vi "Alyssa_GlueLines.vi"() -> ()   [LabVIEW 2016]
uses:
  C:/Users/Aerotech/Documents/BNLStaveAssembly-blueprint/Bin/Aerotech.A3200.dll
  BNLStaveAssembly-blueprint/Bin/Aerotech.A3200.dll
  <vilib>/vision/Image Controls.llb/IMAQ Image.ctl
  <vilib>/LabVIEW Interface for Arduino/Type Defs/Arduino Resource.ctl
  <vilib>/LabVIEW Interface for Arduino/Type Defs/Board Type.ctl
  <vilib>/LabVIEW Interface for Arduino/Type Defs/Pin Mode.ctl
  <vilib>/LabVIEW Interface for Arduino/LabVIEW Interface for Arduino.lvlib
panel:
  out "Module Start":T1
  in  "How many SHORT lines? (actual # will be x2)":i32
  out "XYZ .NET Refnum out 2":refnum<k24>
  in  "y dist (mm)":dbl
  in  "How many lines? (actual # will be x2)":i32
  out "XYZ .NET Refnum out":refnum<k24>
  in  "?":T2(tab)
  in  "Module corner coordinates":T3={"X [mm]"=-325.4922095457569, "Y [mm]"=111.42987050829626, "Z [mm] "=34.99996599632762}
  in  "Axis speeds (mm/s)":T4={"vX [mm]"=49.0, "vY [mm]"=49.0, "vZ [mm] "=49.0}
  in  "Home?":bool
  in  "Lowest Z Position":dbl=38.0
  out "Arduino Resource":T5={"VISA resource"="GlueCTRL", "Board Type"=enum."Uno", "Connection Type"=enum."USB / Serial", "Bytes Per Packet (15)"=15}
  in  "Digital I/O Pin":u8=7
  in  "XYZ Stage Control":refnum<k24>
  in  "Testing?":bool
  out "Difference camera/syringe in X":dbl=-133.03368290747076
  out "Difference camera/syringe in y":dbl=-2.170984960815403
  in  "um/pix resolution":dbl=1.58
  in  "Image Feed":T7=refnum
  in  "Path to save collected images":path=path "C:/Users/Aerotech/cernbox/BNL/Stave Assembly Records/2017-06-12/3"
  in  "Estimate distance y":dbl
  in  "Estimate distance x":dbl=130.0
  in  "Lowest Z position Calibration":dbl=17.0
  out "Final Position":T1={"Final X"=-325.49379764644783, "Final Y"=23.533617154160947, "Final Z"=34.99956596392527}
  out "error out":errorcluster={"status"=FALSE, "code"=1073676418, "source"="VISA Close in GlueSingleModule(SubVI).vi->2_VisualizeModulePositioning2.vi->VMP_TestStand.vi"}
  in  "error in":errorcluster
  # "Timers (ms)"
  # "Overview: This takes a pattern of zeroes/ones (.csv file) as well as the start coordinates of the top left corner of a module and places dots of glue  \nRequirements: NI Arduino dependencies\nInstructions: Select a .csv file (ones indicate regions for glue) as well as a starting coordinate (this is default to the top left corner of the module spacer). You \ncan also input axis speeds (default to maximum) and module lengths and widths (default to 90 mm) which are the widths of the module to which you want to \nplace glue. Lastly, one can choose to Home the stage here and can select the lowest position in Z. The default is that the stage moves down 2-3 mm in Z \nwhile dispensing.  The Arduino inputs are default and simply allow the LabView program to drigger the Arduino (which sends a signal to the dispenser). The \nprogram signals to dispense air- all other parameters such as length of dispensing (default: 350 millisec), pressure (default: 48 psi), and vacuum pressure \n(default: 7.8 psi) are set on the dispenser itself. The defaults are highly recommended here."
  # "Positioning Inputs"
  # "Arduino Inputs"
types:
  T1 = cluster{"Final X":dbl, "Final Y":dbl, "Final Z":dbl}
  T2 = enum32{"Instructions and inputs", "Review  and Error Handling"}
  T3 = cluster{"X [mm]":dbl, "Y [mm]":dbl, "Z [mm] ":dbl}
  T4 = cluster{"vX [mm]":dbl, "vY [mm]":dbl, "vZ [mm] ":dbl}
  T5 = typedef "LabVIEW Interface for Arduino.lvlib/Arduino Resource.ctl" = cluster{"VISA resource":refnum<visa-resource-name>, "Board Type":T6, "Connection Type":enum8{"USB / Serial"}, "Bytes Per Packet (15)":u8}
  T6 = typedef "LabVIEW Interface for Arduino.lvlib/Board Type.ctl" = enum16{"Uno", "Dimuelanove w/Atmega 328", "Mega 2560"}
  T7 = typedef "IMAQ Image.ctl" = refnum<image>
  T8 = typedef "LabVIEW Interface for Arduino.lvlib/Pin Mode.ctl" = enum8{"Input", "Output"}
  T9 = cluster{dbl, "Y [mm]":dbl, "Lowest Z Position":dbl}
  T10 = cluster{"Final X":dbl, "Final Y":dbl, "vZ [mm]":dbl}
  T11 = cluster{"Final X":dbl, "Final Y":dbl, "Lowest Z Position":dbl}
  T12 = cluster{dbl, "Final Y":dbl, "Lowest Z Position":dbl}
  T13 = cluster{"Final X":dbl, "Final Y":dbl, "Z [mm] ":dbl}
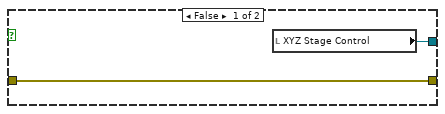
[diagram p2: hidden frame]
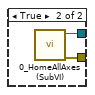
[diagram p3: hidden frame]
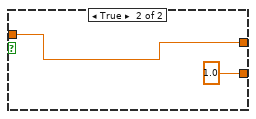
[diagram p5: hidden frame]
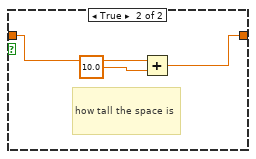
[diagram p6: hidden frame]
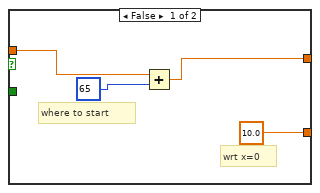
[diagram p7: hidden frame]
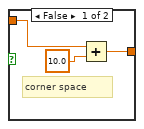
[diagram p8: hidden frame]
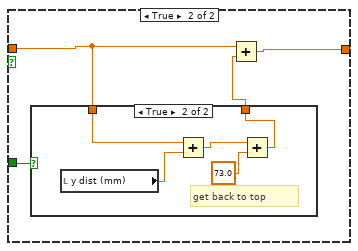
[diagram p9: hidden frame]
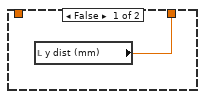
[diagram p10: hidden frame]
diagram:
  n1 = case shown="True" "Testing?" {
    tunnel: [w9 w11] -> w3
    tunnel: [w8 w10] -> w5
    tunnel: "error in" -> [w8 _]
    frame False {
      n2 = local read "XYZ Stage Control"() -> (w9:refnum<k24>)
    }
    frame True {
      n3 = case shown="False" "Home?" {
        tunnel: [w15 w21] -> w11
        tunnel: [w14 w20] -> w10
        frame False {
          w17 = string[] ["X", "Y", "Z"] ("Axes Names")
          n4 = call "Connect.vi"() -> ("error out"=w18:errorcluster, "controller"=w13:refnum<k24>)  [unwired: 10 in]
          n5 = call "EnableMultiple.vi"("error in (no error)"=w18, "axis names"=w17, "controller in"=w13) -> ("error out"=w19:errorcluster, "controller out"=w16:refnum<k24>)  [unwired: 7 in]
          n6 = call "GetCurrentXYZPosition (SubVI).vi"(".NET Refnum in - Device"=w16, "error in (no error)"=w19, "Axes Names"=w17) -> ("error out"=w14:errorcluster, ".NET Refnum out  - Device"=w15:refnum<k24>)  [unwired: 3 in, 4 out]
        }
        frame True {
          n7 = call "0_HomeAllAxes (SubVI).vi"() -> ("error out"=w20:errorcluster, "controller out"=w21:refnum<k24>)  [unwired: 8 in, 2 out]
        }
      }
    }
  }
  n8 = flat-sequence {
    tunnel: [w39] -> w7
    tunnel: w5 -> [w29]
    tunnel: w3 -> [w23]
    tunnel: w7 -> [w192]
    tunnel: [w186] -> w2
    tunnel: w2 -> [w319]
    tunnel: [w318] -> w1
    tunnel: w1 -> [w332]
    frame #0 {
      n9 = flat-sequence {
        tunnel: w29 -> [w53]
        tunnel: [w52] -> w24
        tunnel: w23 -> [w46]
        tunnel: w24 -> [w55]
        tunnel: [w54] -> w22
        tunnel: [w74] -> w26
        tunnel: w22 -> [w73]
        tunnel: w26 -> [w134]
        tunnel: [w132] -> w25
        tunnel: [w165] -> w27
        tunnel: w25 -> [w166]
        frame #0 {
          n10 = local read "Module corner coordinates"() -> (w48:T3)
          n11 = Unbundle(w48) -> ("X [mm]"=w45:dbl, "Y [mm]"=w42:dbl)  [unwired: 1 out]
          n12 = local read "Axis speeds (mm/s)"() -> (w51:T4)
          n13 = Add(x=w45, y=133.0) -> (x+y=w43:dbl)
          n14 = Bundle(w43, "Y [mm]"=w42, "Lowest Z Position"="Lowest Z Position") -> (w47:T9)  [unwired: 1 in]
          n15 = Bundle(w43, "Y [mm]"=w42, "Lowest Z Position"="Lowest Z Position") -> (w40:T9)  [unwired: 1 in]
          n16 = call "Go2XYZ (SubVI).vi"(".NET Refnum in"=w46, "Go to Coordinates"=w47, "Axis Speeds"=w51, "error in (no error)"=w53) -> (".NET Refnum out"=w50:refnum<k24>, "Final Position"=→"Final Position":T1, "error out"=w52:errorcluster)  [unwired: 7 in, 2 out]
          n17 = local write "Module corner coordinates"(w40) -> ()
          n18 = local write "XYZ Stage Control"(w50) -> ()
        }
        frame #1 {
          n19 = while {
            tunnel: w55 -> [w72]
            tunnel: [w68] -> w54
            stop <- w71 stop-if-true
            n20 = local read "Module corner coordinates"() -> (w66:T3)
            n21 = call "Lower glue mount"("error in (no error)"=w72) -> ("Move Z down"=w63:dbl, "Move Z up"=w62:dbl, "Accept current Z?"=w71:bool, "error out"=w69:errorcluster)  [unwired: 14 in, 1 out]
            n22 = local read "Lowest Z Position"() -> (w56:dbl)
            n23 = local read "Axis speeds (mm/s)"() -> (w70:T4)
            n24 = local read "XYZ Stage Control"() -> (w58:refnum<k24>)
            n25 = Add(x=w56, y=w63) -> (x+y=w60:dbl)
            n26 = Subtract(x=w60, y=w62) -> (x-y=w59:dbl)
            n27 = Unbundle(w66) -> ("X [mm]"=w65:dbl, "Y [mm]"=w64:dbl)  [unwired: 1 out]
            n28 = Bundle("X [mm]"=w65, "Y [mm]"=w64, w59) -> (w61:cluster{"X [mm]":dbl, "Y [mm]":dbl, dbl})  [unwired: 1 in]
            n29 = local write "Lowest Z Position"(w59) -> ()
            n30 = call "Go2XYZ (SubVI).vi"(".NET Refnum in"=w58, "Go to Coordinates"=w61, "Axis Speeds"=w70, "error in (no error)"=w69) -> (".NET Refnum out"=w67:refnum<k24>, "Final Position"=w57:T1, "error out"=w68:errorcluster)  [unwired: 7 in, 2 out]
            n31 = local write "XYZ Stage Control"(w67) -> ()
            n32 = local write "Final Position"(w57) -> ()
          }
        }
        frame #2 {
          n33 = call "Calibrate distance?"("error in (no error)"=w73) -> ("Calibrate distance?"=w75:bool, "error out"=w76:errorcluster)  [unwired: 16 in, 1 out]
          n34 = case shown="True" w75 {
            tunnel: w76 -> [w77 w79]
            tunnel: [w77 w80] -> w74
            frame False {
            }
            frame True {
              n35 = flat-sequence {
                tunnel: w79 -> [w82]
                tunnel: [w81] -> w78
                frame #0 {
                  n36 = local read "Final Position"() -> (w89:T1)
                  n37 = local read "Axis speeds (mm/s)"() -> (w85:T4)
                  n38 = local read "XYZ Stage Control"() -> (w84:refnum<k24>)
                  n39 = Unbundle(w89) -> ("Final X"=w87:dbl, "Final Y"=w88:dbl)  [unwired: 1 out]
                  n40 = Bundle("Final X"=w87, "Final Y"=w88, "vZ [mm]"=-20.0) -> (w91:T10)  [unwired: 1 in]
                  n41 = call "Go2XYZ (SubVI).vi"(".NET Refnum in"=w84, "Go to Coordinates"=w91, "Axis Speeds"=w85, "error in (no error)"=w82) -> (".NET Refnum out"=w83:refnum<k24>, "Final Position"=w86:T1, "error out"=w81:errorcluster)  [unwired: 7 in, 2 out]
                  n42 = local write "XYZ Stage Control"(w83) -> ()
                  n43 = local write "Final Position"(w86) -> ()
                }
              }
              n44 = while {
                tunnel: [w130] -> w80
                tunnel: w78 -> [w118]
                i -> [w115]
                stop <- w131 stop-if-true
                n45 = local read "Final Position"() -> (w92:T1)
                n46 = Unbundle(w92) -> ("Final X"=w97:dbl, "Final Y"=w95:dbl, "Final Z"=w96:dbl)
                n47 = local read "Testing?"() -> (w113:bool)
                n48 = local read "Axis speeds (mm/s)"() -> (w120:T4)
                n49 = local read "XYZ Stage Control"() -> (w116:refnum<k24>)
                n50 = Subtract(x=w95, y=220.0) -> (x-y=w93:dbl)
                n51 = Equal To 0?(x=w115) -> (x = 0?=w114:bool)
                n52 = And(x=w113, y=w114) -> (x .and. y?=w112:bool)
                n53 = Bundle("Final X"=w97, w93, "Final Z"=w96) -> (w98:cluster{"Final X":dbl, dbl, "Final Z":dbl})  [unwired: 1 in]
                n54 = call "CalibrateDistanceCameraSyringe.vi"("Path to save collected images"="Path to save collected images", "Image Feed"="Image Feed", "Off stave position"=w98, ".NET Refnum in"=w116, "Axis speeds (mm/s)"=w120, "Lowest Z Position"="Lowest Z position Calibration", "Estimate distance y"="Estimate distance y", "um/pix resolution"="um/pix resolution", "Estimate distance x"="Estimate distance x", "error in"=w118, "Testing?"=w112) -> ("XYZ .NET Refnum out"=w119:refnum<k24>, "error out"=w117:errorcluster, "X/Y difference (CAMERA - SYRINGE)"=w127:dbl[][])  [unwired: 2 in]
                n55 = local read "Difference camera/syringe in X"() -> (w102:dbl)
                n56 = local read "Difference camera/syringe in y"() -> (w99:dbl)
                n57 = local read "Lowest Z position Calibration"() -> (w104:dbl)
                n58 = call "Accept calibration?"("error in (no error)"=w117) -> ("Change in lowest Z"=w106:dbl, "Change in distance Y estimate"=w107:dbl, "Change in distance X estimate"=w108:dbl, "Accept the distance syringe/camera?"=w131:bool, "error out"=w130:errorcluster)  [unwired: 13 in, 1 out]
                n59 = local write "XYZ Stage Control"(w119) -> ()
                n60 = Index Array(array=w127, index (row) #1=0 ("index (row)"), index (col) #1=0 ("disabled index (col)"), index (row) #2=0 ("index (row)"), index (col) #2=1 ("disabled index (col)")) -> (element #1=→"Difference camera/syringe in X":dbl, element #2=→"Difference camera/syringe in y":dbl)
                n61 = Add(x=w102, y=w108) -> (x+y=w101:dbl)
                n62 = Add(x=w99, y=w107) -> (x+y=w100:dbl)
                n63 = Add(x=w104, y=w106) -> (x+y=w105:dbl)
                n64 = local write "Difference camera/syringe in X"(w101) -> ()
                n65 = local write "Difference camera/syringe in y"(w100) -> ()
                n66 = local write "Lowest Z position Calibration"(w105) -> ()
              }
            }
          }
        }
        frame #3 {
          n67 = flat-sequence {
            tunnel: w134 -> [w141]
            tunnel: [w138] -> w133
            tunnel: [w152] -> w132
            tunnel: w133 -> [w153]
            frame #0 {
              n68 = local read "Module corner coordinates"() -> (w151:T3)
              n69 = local read "Difference camera/syringe in y"() -> (w146:dbl)
              n70 = local read "Difference camera/syringe in X"() -> (w147:dbl)
              n71 = Unbundle By Name(w151) -> ("X [mm]"=w137:dbl, "Y [mm]"=w150:dbl)  [unwired: 1 out]
              n72 = Subtract(x=w150, y=w146) -> (x-y=w148:dbl)
              n73 = Subtract(x=w137, y=133.0) -> (x-y=w135:dbl)
              n74 = local read "Axis speeds (mm/s)"() -> (w142:T4)
              n75 = local read "XYZ Stage Control"() -> (w143:refnum<k24>)
              n76 = Subtract(x=w135, y=w147) -> (x-y=w149:dbl)
              n77 = Bundle(w149, w148, "index (row)"=-20.0) -> (w140:cluster{dbl, dbl, "index (row)":dbl})  [unwired: 1 in]
              n78 = call "Go2XYZ (SubVI).vi"(".NET Refnum in"=w143, "Go to Coordinates"=w140, "Axis Speeds"=w142, "error in (no error)"=w141) -> (".NET Refnum out"=w144:refnum<k24>, "Final Position"=w145:T1, "error out"=w138:errorcluster)  [unwired: 7 in, 2 out]
              n79 = local write "XYZ Stage Control"(w144) -> ()
              n80 = local write "Module corner coordinates"(w145) -> ()
            }
            frame #1 {
              n81 = local read "Module corner coordinates"() -> (w158:T3)
              n82 = local read "Lowest Z Position"() -> (w161:dbl)
              n83 = local read "Axis speeds (mm/s)"() -> (w155:T4)
              n84 = local read "XYZ Stage Control"() -> (w154:refnum<k24>)
              n85 = Unbundle(w158) -> ("X [mm]"=w159:dbl, "Y [mm]"=w160:dbl)  [unwired: 1 out]
              n86 = Subtract(x=w161, y=2.0) -> (x-y=w163:dbl)
              n87 = Bundle("X [mm]"=w159, "Y [mm]"=w160, w163) -> (w164:cluster{"X [mm]":dbl, "Y [mm]":dbl, dbl})  [unwired: 1 in]
              n88 = call "Go2XYZ (SubVI).vi"(".NET Refnum in"=w154, "Go to Coordinates"=w164, "Axis Speeds"=w155, "error in (no error)"=w153) -> (".NET Refnum out"=w156:refnum<k24>, "Final Position"=w157:T1, "error out"=w152:errorcluster)  [unwired: 7 in, 2 out]
              n89 = local write "XYZ Stage Control"(w156) -> ()
              n90 = local write "Module corner coordinates"(w157) -> ()
            }
          }
        }
        frame #4 {
          n91 = while {
            tunnel: w166 -> [w180]
            tunnel: [w182] -> w165
            stop <- w167 continue-if-true
            n92 = local read "Module corner coordinates"() -> (w179:T3)
            n93 = call "Ready to glue?"("error in (no error)"=w180) -> ("Move in Z"=w176:dbl, "Move in Y"=w177:dbl, "Move in X"=w178:dbl, "Oh yeah! Reset Arduino and go!"=w167:bool, "error out"=w181:errorcluster)  [unwired: 13 in, 1 out]
            n94 = local read "Axis speeds (mm/s)"() -> (w185:T4)
            n95 = local read "XYZ Stage Control"() -> (w183:refnum<k24>)
            n96 = Unbundle(w179) -> ("X [mm]"=w175:dbl, "Y [mm]"=w174:dbl, "Z [mm]"=w173:dbl)
            n97 = Add(x=w175, y=w178) -> (x+y=w170:dbl)
            n98 = Add(x=w174, y=w177) -> (x+y=w172:dbl)
            n99 = Add(x=w173, y=w176) -> (x+y=w171:dbl)
            n100 = Bundle(w170, w172, w171) -> (w169:cluster{dbl, dbl, dbl})  [unwired: 1 in]
            n101 = call "Go2XYZ (SubVI).vi"(".NET Refnum in"=w183, "Go to Coordinates"=w169, "Axis Speeds"=w185, "error in (no error)"=w181) -> (".NET Refnum out"=w184:refnum<k24>, "Final Position"=w168:T1, "error out"=w182:errorcluster)  [unwired: 7 in, 2 out]
            "Module Start" <- w168
            n102 = local write "XYZ Stage Control"(w184) -> ()
            n103 = local write "Final Position"(w168) -> ()
            n104 = local write "Module corner coordinates"(w168) -> ()
          }
        }
      }
      n105 = local read "Digital I/O Pin"() -> (w28:u8)
      n106 = call <vilib>:"Init.vi"("VISA resource"=refnum<visa-resource-name> "GlueCTRL", "error in"=w27) -> ("Arduino Resource"=w31:T5, "error out"=w32:errorcluster)  [unwired: 16 in]
      "Arduino Resource" <- w31
      n107 = call <vilib>:"Set Digital Pin Mode.vi"("Arduino Resource"=w31, "Digital I/O Pin"="Digital I/O Pin", "Pin Mode (Input)"=Pin_Mode."Output", "error in"=w32) -> ("Arduino Resource"=w35:T5, "error out"=w36:errorcluster)  [unwired: 10 in]
      n108 = call <vilib>:"Digital Write Pin.vi"("Arduino Resource"=w35, "Digital I/O Pin (0)"=w28, "Value (0)"=u8 0, "error in"=w36) -> ("Arduino Resource"=w30:T5, "error out"=w39:errorcluster)  [unwired: 10 in]
      n109 = local write "Arduino Resource"(w30) -> ()
    }
    frame #1 {
      (unwired) u8 0 ("Value (0)")
      n110 = local read "Module Start"() -> (w191:T1)
      n111 = Unbundle By Name(w191) -> ("Final X"=w189:dbl, "Final Y"=w188:dbl, "Final Z"=w187:dbl)
      n112 = for {
        N: "How many lines? (actual # will be x2)" -> [_]
        tunnel: w192 -> [w207]
        tunnel: [w206] -> w186
        shift-right: [w204] -> _
        shift-left: w188 -> [w205]
        tunnel: w187 -> [w203]
        shift-right: [w202] -> _
        shift-left: w189 -> [w201]
        i -> [w194]
        n113 = local read "How many lines? (actual # will be x2)"() -> (w197:i32)
        n114 = Subtract(x=w197, y=2) -> (x-y=w195:i32)
        n115 = Equal?(x=w194, y=w195) -> (x = y?=w193:bool)
        n116 = Equal To 0?(x=w194) -> (x = 0?=w199:bool)
        n117 = Or(x=w199, y=w193) -> (x .or. y?=w198:bool)
        n118 = for {
          N: 2 -> [_]
          tunnel: w207 -> [w231]
          tunnel: [w229] -> w206
          shift-right: [w228] -> w204
          shift-left: w205 -> [w218]
          tunnel: w198 -> [w219]
          tunnel: w203 -> [w217]
          tunnel: w201 -> [w220]
          tunnel: [w215] -> w202
          i -> [w216]
          n119 = flat-sequence {
            tunnel: w231 -> [w247]
            tunnel: [w237] -> w226
            tunnel: [w247] -> w225
            tunnel: [w238] -> w224
            tunnel: [w236] -> w223
            tunnel: [w240] -> w222
            tunnel: [w238] -> w221
            tunnel: w220 -> [w235]
            tunnel: w219 -> [w234]
            tunnel: w218 -> [w241]
            tunnel: w217 -> [w240]
            tunnel: w216 -> [w239]
            tunnel: [w260] -> w213
            tunnel: [w264] -> w211
            tunnel: [w261] -> w209
            tunnel: w226 -> [w260]
            tunnel: w225 -> [w265]
            tunnel: w224 -> [w270]
            tunnel: w223 -> [w271]
            tunnel: w222 -> [w269]
            tunnel: w221 -> [w261]
            tunnel: w213 -> [w283]
            tunnel: [w283] -> w212
            tunnel: w211 -> [w282]
            tunnel: [w282] -> w210
            tunnel: w209 -> [w281]
            tunnel: [w281] -> w208
            tunnel: [w297] -> w233
            tunnel: [w296] -> w232
            tunnel: [w295] -> w230
            tunnel: [w287] -> w227
            tunnel: w212 -> [w285]
            tunnel: w210 -> [w284]
            tunnel: w208 -> [w287]
            tunnel: [w285] -> w214
            tunnel: [w317] -> w229
            tunnel: w230 -> [w302]
            tunnel: w232 -> [w316]
            tunnel: w233 -> [w314]
            tunnel: [w301] -> w228
            tunnel: w227 -> [w301]
            tunnel: [w300] -> w215
            tunnel: w214 -> [w300]
            frame #0 {
              # "line length"
              n120 = Equal To 0?(x=w239) -> (x = 0?=w246:bool)
              n121 = And(x=w246, y=w234) -> (x .and. y?=w245:bool)
              n122 = case shown="False" w246 {
                tunnel: [0.0 1.0] -> w244
                tunnel: [w249 w252] -> w236
                tunnel: w235 -> [w250 w252]
                frame False {
                  # "start @ end of line"
                  n123 = Add(x=w250, y=85 ("x")) -> (x+y=w249:dbl)
                }
                frame True {
                }
              }
              n124 = case shown="False" w245 {
                tunnel: w241 -> [w256 w259]
                tunnel: [w255 w258] -> w238
                frame False {
                  n125 = Add(x=w256, y="y dist (mm)") -> (x+y=w255:dbl)
                }
                frame True {
                  # "how tall the space is"
                  n126 = Add(x=w259, y=10.0) -> (x+y=w258:dbl)
                }
              }
              n127 = Multiply(x=85, y=w244) -> (x*y=w243:dbl)
              n128 = Add(x=w235, y=w243) -> (x+y=w237:dbl)
            }
            frame #1 {
              n129 = local read "Axis speeds (mm/s)"() -> (w267:T4)
              n130 = local read "XYZ Stage Control"() -> (w263:refnum<k24>)
              n131 = Bundle("Final X"=w271, w270, "Final Z"=w269) -> (w268:cluster{"Final X":dbl, dbl, "Final Z":dbl})  [unwired: 1 in]
              n132 = call "Go2XYZ (SubVI).vi"(".NET Refnum in"=w263, "Go to Coordinates"=w268, "Axis Speeds"=w267, "error in (no error)"=w265) -> (".NET Refnum out"=w262:refnum<k24>, "Final Position"=w266:T1, "error out"=w264:errorcluster)  [unwired: 7 in, 2 out]
              n133 = local write "XYZ Stage Control"(w262) -> ()
              n134 = local write "Final Position"(w266) -> ()
            }
            frame #2 {
              n135 = local read "XYZ Stage Control"() -> (w280:refnum<k24>)
              n136 = local read "Final Position"() -> (w276:T1)
              n137 = Unbundle(w276) -> ("Final X"=w275:dbl, "Final Y"=w274:dbl)  [unwired: 1 out]
              n138 = local read "Lowest Z Position"() -> (w273:dbl)
              n139 = Bundle("Final X"=w275, "Final Y"=w274, "Lowest Z Position"=w273) -> (w272:T11)  [unwired: 1 in]
              n140 = local read "Axis speeds (mm/s)"() -> (w277:T4)
              n141 = call "Go2XYZ (SubVI).vi"(".NET Refnum in"=w280, "Go to Coordinates"=w272, "Axis Speeds"=w277) -> (".NET Refnum out"=w279:refnum<k24>, "Final Position"=w278:T1)  [unwired: 8 in, 3 out]
              n142 = local write "XYZ Stage Control"(w279) -> ()
              n143 = local write "Final Position"(w278) -> ()
            }
            frame #3 {
              n144 = local read "Final Position"() -> (w288:T1)
              n145 = local read "Arduino Resource"() -> (w298:T5)
              n146 = local read "Lowest Z Position"() -> (w294:dbl)
              n147 = local read "Digital I/O Pin"() -> (w297:u8)
              n148 = local read "Axis speeds (mm/s)"() -> (w291:T4)
              n149 = local read "XYZ Stage Control"() -> (w292:refnum<k24>)
              n150 = Unbundle(w288) -> ("Final Y"=w286:dbl)  [unwired: 2 out]
              n151 = Bundle(w285, "Final Y"=w286, "Lowest Z Position"=w294) -> (w290:T12)  [unwired: 1 in]
              n152 = call <vilib>:"Digital Write Pin.vi"("Arduino Resource"=w298, "Digital I/O Pin (0)"=w297, "Value (0)"=u8 1, "error in"=w284) -> ("Arduino Resource"=w296:T5, "error out"=w295:errorcluster)  [unwired: 10 in]
              n153 = call "Go2XYZ (SubVI).vi"(".NET Refnum in"=w292, "Go to Coordinates"=w290, "Axis Speeds"=w291) -> (".NET Refnum out"=w293:refnum<k24>, "Final Position"=w289:T1)  [unwired: 8 in, 3 out]
              n154 = local write "Arduino Resource"(w296) -> ()
              n155 = local write "XYZ Stage Control"(w293) -> ()
              n156 = local write "Final Position"(w289) -> ()
            }
            frame #4 {
              n157 = local read "Module corner coordinates"() -> (w311:T3)
              n158 = call <vilib>:"Digital Write Pin.vi"("Arduino Resource"=w316, "Digital I/O Pin (0)"=w314, "Value (0)"=u8 0, "error in"=w302) -> ("Arduino Resource"=w313:T5, "error out"=w317:errorcluster)  [unwired: 10 in]
              n159 = local write "Arduino Resource"(w313) -> ()
              n160 = local read "Final Position"() -> (w312:T1)
              n161 = local read "Axis speeds (mm/s)"() -> (w306:T4)
              n162 = local read "XYZ Stage Control"() -> (w305:refnum<k24>)
              n163 = Unbundle(w312) -> ("Final X"=w310:dbl, "Final Y"=w309:dbl)  [unwired: 1 out]
              n164 = Unbundle(w311) -> ("Z [mm]"=w308:dbl)  [unwired: 2 out]
              n165 = Bundle("Final X"=w310, "Final Y"=w309, "Z [mm]"=w308) -> (w307:T13)  [unwired: 1 in]
              n166 = call "Go2XYZ (SubVI).vi"(".NET Refnum in"=w305, "Go to Coordinates"=w307, "Axis Speeds"=w306) -> (".NET Refnum out"=→"XYZ .NET Refnum out":refnum<k24>, "Final Position"=w304:T1)  [unwired: 8 in, 3 out]
              n167 = local write "Final Position"(w304) -> ()
            }
          }
        }
      }
    }
    frame #2 {
      n168 = call "Phase Two!"("error in (no error)"=w319) -> ("error out"=w318:errorcluster)  [unwired: 16 in, 2 out]
    }
    frame #3 {
      n169 = local read "Module Start"() -> (w333:T1)
      n170 = Unbundle By Name(w333) -> ("Final X"=w320:dbl, "Final Y"=w321:dbl, "Final Z"=w330:dbl)
      n171 = for {
        N: "How many SHORT lines? (actual # will be x2)" -> [_]
        tunnel: w332 -> [w348]
        tunnel: [w347] -> w324
        shift-right: [w345] -> _
        shift-left: w321 -> [w346]
        tunnel: w330 -> [w344]
        shift-right: [w343] -> _
        shift-left: w320 -> [w342]
        i -> [w335]
        # "move in x"
        n172 = local read "How many SHORT lines? (actual # will be x2)"() -> (w338:i32)
        n173 = Subtract(x=w338, y=1) -> (x-y=w336:i32)
        n174 = Equal?(x=w335, y=w336) -> (x = y?=w334:bool)
        n175 = Equal To 0?(x=w335) -> (x = 0?=w340:bool)
        n176 = Or(x=w340, y=w334) -> (x .or. y?=w339:bool)
        n177 = for {
          N: 2 -> [_]
          tunnel: w348 -> [w370]
          tunnel: [w368] -> w347
          shift-right: [w367] -> w345
          shift-left: w346 -> [w357]
          tunnel: w339 -> [w358]
          tunnel: w344 -> [w356]
          tunnel: w342 -> [w359]
          tunnel: [w354] -> w343
          tunnel: w334 -> [w352]
          i -> [w355]
          # "move in y"
          n178 = flat-sequence {
            tunnel: w370 -> [w385]
            tunnel: [w378] -> w365
            tunnel: [w385] -> w364
            tunnel: [w379] -> w363
            tunnel: [w377] -> w362
            tunnel: [w381] -> w361
            tunnel: [w379] -> w360
            tunnel: w359 -> [w376]
            tunnel: w358 -> [w374]
            tunnel: w357 -> [w382]
            tunnel: w356 -> [w381]
            tunnel: w355 -> [w380]
            tunnel: w352 -> [w373]
            tunnel: [w422] -> w351
            tunnel: [w421] -> w350
            tunnel: [w420] -> w349
            tunnel: w360 -> [w420]
            tunnel: w361 -> [w417]
            tunnel: w362 -> [w419]
            tunnel: w363 -> [w418]
            tunnel: w364 -> [w413]
            tunnel: w365 -> [w422]
            tunnel: [w436] -> w372
            tunnel: [w435] -> w371
            tunnel: [w434] -> w369
            tunnel: [w426] -> w366
            tunnel: w351 -> [w424]
            tunnel: w350 -> [w423]
            tunnel: w349 -> [w426]
            tunnel: [w424] -> w353
            tunnel: [w456] -> w368
            tunnel: w369 -> [w441]
            tunnel: w371 -> [w455]
            tunnel: w372 -> [w453]
            tunnel: [w440] -> w367
            tunnel: w366 -> [w440]
            tunnel: [w439] -> w354
            tunnel: w353 -> [w439]
            frame #0 {
              # "where to move"
              n179 = Equal To 0?(x=w380) -> (x = 0?=w384:bool)
              n180 = And(x=w384, y=w374) -> (x .and. y?=w383:bool)
              n181 = case shown="False" w383 {
                tunnel: w382 -> [w400 w401]
                tunnel: [w399 w404] -> w379
                tunnel: w373 -> [_ w403]
                frame False {
                  n182 = local read "y dist (mm)"() -> (w398:dbl)
                  n183 = Subtract(x=w400, y=w398) -> (x-y=w399:dbl)
                }
                frame True {
                  n184 = case shown="True" w403 {
                    tunnel: [w405 w406] -> w402
                    tunnel: w401 -> [_ w409]
                    frame False {
                      n185 = local read "y dist (mm)"() -> (w405:dbl)
                    }
                    frame True {
                      # "get back to top"
                      n186 = local read "y dist (mm)"() -> (w410:dbl)
                      n187 = Add(x=w409, y=w410) -> (x+y=w408:dbl)
                      n188 = Add(x=w408, y=73.0) -> (x+y=w406:dbl)
                    }
                  }
                  n189 = Add(x=w401, y=w402) -> (x+y=w404:dbl)
                }
              }
              n190 = case shown="True" w384 {
                tunnel: [w388 w392] -> w377
                tunnel: w376 -> [w389 w393]
                tunnel: w373 -> [_ w391]
                tunnel: [10.0 65.0 ("y")] -> w375
                frame False {
                  # "wrt x=0"
                  # "where to start"
                  n191 = Add(x=w389, y=65 ("x")) -> (x+y=w388:dbl)
                }
                frame True {
                  # "where to start"
                  n192 = case shown="True" w391 {
                    tunnel: w393 -> [w396 w397]
                    tunnel: [w395 w397] -> w392
                    frame False {
                      # "corner space"
                      n193 = Add(x=w396, y=10.0) -> (x+y=w395:dbl)
                    }
                    frame True {
                    }
                  }
                }
              }
              n194 = Add(x=w376, y=w375) -> (x+y=w378:dbl)
            }
            frame #1 {
              n195 = local read "Axis speeds (mm/s)"() -> (w415:T4)
              n196 = local read "XYZ Stage Control"() -> (w412:refnum<k24>)
              n197 = Bundle("Final X"=w419, w418, "Final Z"=w417) -> (w416:cluster{"Final X":dbl, dbl, "Final Z":dbl})  [unwired: 1 in]
              n198 = call "Go2XYZ (SubVI).vi"(".NET Refnum in"=w412, "Go to Coordinates"=w416, "Axis Speeds"=w415, "error in (no error)"=w413) -> (".NET Refnum out"=w411:refnum<k24>, "Final Position"=w414:T1, "error out"=w421:errorcluster)  [unwired: 7 in, 2 out]
              n199 = local write "XYZ Stage Control"(w411) -> ()
              n200 = local write "Final Position"(w414) -> ()
            }
            frame #2 {
              n201 = local read "Final Position"() -> (w427:T1)
              n202 = local read "Arduino Resource"() -> (w437:T5)
              n203 = local read "Lowest Z Position"() -> (w433:dbl)
              n204 = local read "Digital I/O Pin"() -> (w436:u8)
              n205 = local read "Axis speeds (mm/s)"() -> (w430:T4)
              n206 = local read "XYZ Stage Control"() -> (w431:refnum<k24>)
              n207 = Unbundle(w427) -> ("Final Y"=w425:dbl)  [unwired: 2 out]
              n208 = Bundle(w424, "Final Y"=w425, "Lowest Z Position"=w433) -> (w429:T12)  [unwired: 1 in]
              n209 = call <vilib>:"Digital Write Pin.vi"("Arduino Resource"=w437, "Digital I/O Pin (0)"=w436, "Value (0)"=u8 1, "error in"=w423) -> ("Arduino Resource"=w435:T5, "error out"=w434:errorcluster)  [unwired: 10 in]
              n210 = call "Go2XYZ (SubVI).vi"(".NET Refnum in"=w431, "Go to Coordinates"=w429, "Axis Speeds"=w430) -> (".NET Refnum out"=w432:refnum<k24>, "Final Position"=w428:T1)  [unwired: 8 in, 3 out]
              n211 = local write "Arduino Resource"(w435) -> ()
              n212 = local write "XYZ Stage Control"(w432) -> ()
              n213 = local write "Final Position"(w428) -> ()
            }
            frame #3 {
              n214 = call <vilib>:"Digital Write Pin.vi"("Arduino Resource"=w455, "Digital I/O Pin (0)"=w453, "Value (0)"=u8 0, "error in"=w441) -> ("Arduino Resource"=w452:T5, "error out"=w456:errorcluster)  [unwired: 10 in]
              n215 = local read "Module Start"() -> (w450:T1)
              n216 = local write "Arduino Resource"(w452) -> ()
              n217 = local read "Final Position"() -> (w451:T1)
              n218 = local read "Axis speeds (mm/s)"() -> (w445:T4)
              n219 = local read "XYZ Stage Control"() -> (w444:refnum<k24>)
              n220 = Unbundle(w451) -> ("Final X"=w449:dbl, "Final Y"=w448:dbl)  [unwired: 1 out]
              n221 = Unbundle(w450) -> ("Final Z"=w447:dbl)  [unwired: 2 out]
              n222 = Bundle("Final X"=w449, "Final Y"=w448, "Final Z"=w447) -> (w446:T1)  [unwired: 1 in]
              n223 = call "Go2XYZ (SubVI).vi"(".NET Refnum in"=w444, "Go to Coordinates"=w446, "Axis Speeds"=w445) -> (".NET Refnum out"=→"XYZ .NET Refnum out 2":refnum<k24>, "Final Position"=w443:T1)  [unwired: 8 in, 3 out]
              n224 = local write "Final Position"(w443) -> ()
            }
          }
        }
      }
      n225 = local read "Arduino Resource"() -> (w323:T5)
      n226 = local read "Digital I/O Pin"() -> (w322:u8)
      n227 = call <vilib>:"Digital Write Pin.vi"("Arduino Resource"=w323, "Digital I/O Pin (0)"=w322, "error in"=w324) -> ("Arduino Resource"=w328:T5, "error out"=w327:errorcluster)  [unwired: 11 in]
      n228 = call <vilib>:"Close.vi"("Arduino Resource"=w328, "error in"=w327) -> ("error out"=w326:errorcluster)  [unwired: 13 in]
      n229 = VISA Close(VISA resource name=refnum<visa-resource-name> "COM3", error in (no error)=w326) -> (error out=→"error out":errorcluster)
    }
  }
